vi "Dresden R2R Sputter 03.02.2018 IY24.vi"() -> ()   [LabVIEW 2009] (continued)
                                }
                                frame #1 {
                                }
                                }
                                }
                                frame #2 {
                                n31527 = local read "Semi"() -> (w36220:bool)
                                n31528 = case shown="False" w36220 {
                                frame #0 {
                                n31529 = local write "Dc_auto_set_zero"(TRUE ("Dc_auto_set")) -> ()
                                }
                                frame #1 {
                                }
                                }
                                }
                                frame #3 {
                                n31530 = local read "Semi"() -> (w36222:bool)
                                n31531 = case shown="False" w36222 {
                                frame #0 {
                                n31532 = Wait (ms)(milliseconds to wait=u32 1000) -> ()  [unwired: 1 out]
                                }
                                frame #1 {
                                }
                                }
                                }
                                frame #4 {
                                n31533 = local read "Semi"() -> (w36224:bool)
                                n31534 = case shown="False" w36224 {
                                frame #0 {
                                n31535 = while {
                                i -> [w36236]
                                stop <- w36225 stop-if-true
                                n31536 = Greater?(x=w36236, y=600) -> (0:w36235:bool)
                                n31537 = case shown="True" w36235 {
                                frame #0 {
                                }
                                frame #1 {
                                n31538 = local write "Semi"(TRUE ("Semi")) -> ()
                                n31539 = local write "Error Message"("Sputter Process cancelled.\nPlease Check DC connections." ("Error Message")) -> ()
                                }
                                }
                                n31540 = local read "Actual DC Power"() -> (w36230:dbl)
                                n31541 = local read "Actual DC Volt :"() -> (w36229:dbl)
                                n31542 = Less?(x=w36230, y=10.0) -> (x < y?=w36233:bool)
                                n31543 = Less?(x=w36229, y=20.0) -> (x < y?=w36234:bool)
                                n31544 = And(x=w36233, y=w36234) -> (x .and. y?=w36227:bool)
                                n31545 = local read "Semi"() -> (w36226:bool)
                                n31546 = Wait Until Next ms Multiple(millisecond multiple=u32 500) -> ()  [unwired: 1 out]
                                n31547 = Compound Arithmetic op=OR(w36227, w36226) -> (w36225:bool)
                                }
                                }
                                frame #1 {
                                }
                                }
                                }
                                frame #5 {
                                n31548 = local read "Semi"() -> (w36240:bool)
                                n31549 = case shown="False" w36240 {
                                frame #0 {
                                n31550 = while {
                                i -> [w36246]
                                stop <- w36241 stop-if-true
                                n31551 = Greater?(x=w36246, y=50) -> (0:w36245:bool)
                                n31552 = case shown="True" w36245 {
                                frame #0 {
                                }
                                frame #1 {
                                n31553 = local write "Semi"(TRUE ("Semi")) -> ()
                                n31554 = local write "Error Message"("Sputter Process cancelled.\nPlease Check DCPS-SW1." ("Error Message")) -> ()
                                }
                                }
                                n31555 = local read "Cnt_Dcps_sw1_di"() -> (w36244:bool)
                                n31556 = case shown="True" w36244 {
                                tunnel: [TRUE ("Cnt_Dcps_sw1_do") FALSE ("Cnt_Dcps_sw1_do")] -> w36243
                                frame #0 {
                                }
                                frame #1 {
                                n31557 = local write "Cnt_Dcps_sw1_do"(FALSE ("Cnt_Dcps_sw1_do")) -> ()
                                n31558 = Wait Until Next ms Multiple(millisecond multiple=u32 500) -> ()  [unwired: 1 out]
                                }
                                }
                                n31559 = local read "Semi"() -> (w36242:bool)
                                n31560 = Or(x=w36243, y=w36242) -> (x .or. y?=w36241:bool)
                                }
                                }
                                frame #1 {
                                }
                                }
                                }
                                frame #6 {
                                n31561 = local read "Semi"() -> (w36254:bool)
                                n31562 = case shown="False" w36254 {
                                frame #0 {
                                n31563 = Wait (ms)(milliseconds to wait=u32 1000) -> ()  [unwired: 1 out]
                                n31564 = local write "SDC1 25"(TRUE ("SDC1 25")) -> ()
                                }
                                frame #1 {
                                }
                                }
                                }
                                }
                                }
                                frame #1 {
                                }
                                }
                                }
                                frame #14 {
                                # "PC-BV OPEN"
                                n31565 = stacked-sequence {
                                frame #0 {
                                n31566 = local read "Semi"() -> (w36257:bool)
                                n31567 = case shown="False" w36257 {
                                frame #0 {
                                n31568 = stacked-sequence {
                                frame #0 {
                                n31569 = local read "Semi"() -> (w36258:bool)
                                n31570 = case shown="False" w36258 {
                                frame #0 {
                                n31571 = local write "Pc_bv2_auto_open"(TRUE ("Tp1_auto_start")) -> ()
                                }
                                frame #1 {
                                }
                                }
                                }
                                frame #1 {
                                n31572 = local read "Semi"() -> (w36260:bool)
                                n31573 = case shown="False" w36260 {
                                frame #0 {
                                n31574 = Wait (ms)(milliseconds to wait=u32 1000) -> ()  [unwired: 1 out]
                                }
                                frame #1 {
                                }
                                }
                                }
                                frame #2 {
                                n31575 = local read "Semi"() -> (w36262:bool)
                                n31576 = case shown="False" w36262 {
                                frame #0 {
                                n31577 = while {
                                i -> [w36268]
                                stop <- w36264 stop-if-true
                                n31578 = local read "Pc_bv_opened_ch2"() -> (w36266:bool)
                                n31579 = Greater?(x=w36268, y=120) -> (0:w36267:bool)
                                n31580 = local read "Semi"() -> (w36265:bool)
                                n31581 = Compound Arithmetic op=OR(w36265, w36266, w36267) -> (w36264:bool)
                                n31582 = Wait (ms)(milliseconds to wait=u32 500) -> ()  [unwired: 1 out]
                                }
                                }
                                frame #1 {
                                }
                                }
                                }
                                frame #3 {
                                n31583 = local read "Semi"() -> (w36270:bool)
                                n31584 = case shown="False" w36270 {
                                frame #0 {
                                n31585 = local read "Pc_bv_opened_ch2"() -> (w36271:bool)
                                n31586 = case shown="False" w36271 {
                                frame #0 {
                                n31587 = local write "Pc_bv2_auto_open"(TRUE ("Pc_bv1_auto_open")) -> ()
                                }
                                frame #1 {
                                }
                                }
                                }
                                frame #1 {
                                }
                                }
                                }
                                frame #4 {
                                n31588 = local read "Semi"() -> (w36273:bool)
                                n31589 = case shown="False" w36273 {
                                frame #0 {
                                n31590 = local read "Pc_bv_opened_ch2"() -> (w36274:bool)
                                n31591 = case shown="False" w36274 {
                                frame #0 {
                                n31592 = Wait (ms)(milliseconds to wait=u32 1000) -> ()  [unwired: 1 out]
                                }
                                frame #1 {
                                }
                                }
                                }
                                frame #1 {
                                }
                                }
                                }
                                frame #5 {
                                n31593 = local read "Semi"() -> (w36276:bool)
                                n31594 = case shown="False" w36276 {
                                frame #0 {
                                n31595 = while {
                                i -> [w36282]
                                stop <- w36278 stop-if-true
                                n31596 = local read "Pc_bv_opened_ch2"() -> (w36280:bool)
                                n31597 = Greater?(x=w36282, y=120) -> (0:w36281:bool)
                                n31598 = local read "Semi"() -> (w36279:bool)
                                n31599 = Compound Arithmetic op=OR(w36279, w36280, w36281) -> (w36278:bool)
                                n31600 = Wait (ms)(milliseconds to wait=u32 500) -> ()  [unwired: 1 out]
                                }
                                }
                                frame #1 {
                                }
                                }
                                }
                                frame #6 {
                                n31601 = local read "Semi"() -> (w36284:bool)
                                n31602 = case shown="False" w36284 {
                                frame #0 {
                                n31603 = local read "Pc_bv_opened_ch2"() -> (w36285:bool)
                                n31604 = case shown="False" w36285 {
                                frame #0 {
                                n31605 = local write "Error Message"("Start up process  cancelled\nbecause  PC-BV not opened.\nPlease check PC-BV1 connections." ("Error Message")) -> ()
                                n31606 = Wait (ms)(milliseconds to wait=u32 1000) -> ()  [unwired: 1 out]
                                }
                                frame #1 {
                                }
                                }
                                }
                                frame #1 {
                                }
                                }
                                }
                                }
                                }
                                frame #1 {
                                }
                                }
                                }
                                frame #1 {
                                n31607 = local read "Semi"() -> (w36288:bool)
                                n31608 = case shown="False" w36288 {
                                frame #0 {
                                n31609 = Wait (ms)(milliseconds to wait=u32 1000) -> ()  [unwired: 1 out]
                                n31610 = local write "SDC1 28"(TRUE ("SDC1 28")) -> ()
                                }
                                frame #1 {
                                }
                                }
                                }
                                }
                                }
                                frame #15 {
                                # "set ar zero"
                                n31611 = stacked-sequence {
                                frame #0 {
                                n31612 = local read "Semi"() -> (w36291:bool)
                                n31613 = case shown="False" w36291 {
                                frame #0 {
                                n31614 = stacked-sequence {
                                frame #0 {
                                n31615 = local read "Semi"() -> (w36292:bool)
                                n31616 = case shown="False" w36292 {
                                frame #0 {
                                n31617 = local write "Ar_auto_set_zero_ch2"(TRUE ("Ar_auto_set_zero_ch1")) -> ()
                                }
                                frame #1 {
                                }
                                }
                                }
                                frame #1 {
                                n31618 = local read "Semi"() -> (w36294:bool)
                                n31619 = case shown="False" w36294 {
                                frame #0 {
                                n31620 = while {
                                i -> [w36297]
                                stop <- w36296 stop-if-true
                                n31621 = Greater?(x=w36297, y=150) -> (0:w36296:bool)
                                n31622 = local read "Semi"() -> (w36295:bool)
                                n31623 = case shown="False" w36295 {
                                tunnel: [FALSE TRUE] -> _
                                frame #0 {
                                n31624 = Wait Until Next ms Multiple(millisecond multiple=u32 200) -> ()  [unwired: 1 out]
                                }
                                frame #1 {
                                }
                                }
                                }
                                }
                                frame #1 {
                                }
                                }
                                }
                                frame #2 {
                                n31625 = local read "Semi"() -> (w36302:bool)
                                n31626 = case shown="False" w36302 {
                                frame #0 {
                                n31627 = local read "Ar_sccm_act 6"() -> (w36304:dbl)
                                n31628 = Less?(x=w36304, y=1) -> (x < y?=w36303:bool)
                                n31629 = case shown="False" w36303 {
                                frame #0 {
                                n31630 = local write "Ar_auto_set_zero_ch2"(TRUE ("Ar_auto_set_zero_ch1")) -> ()
                                }
                                frame #1 {
                                }
                                }
                                }
                                frame #1 {
                                }
                                }
                                }
                                frame #3 {
                                n31631 = local read "Semi"() -> (w36307:bool)
                                n31632 = case shown="False" w36307 {
                                frame #0 {
                                n31633 = local read "Ar_sccm_act 6"() -> (w36309:dbl)
                                n31634 = Less?(x=w36309, y=1) -> (x < y?=w36308:bool)
                                n31635 = case shown="False" w36308 {
                                frame #0 {
                                n31636 = while {
                                i -> [w36315]
                                stop <- w36312 stop-if-true
                                n31637 = Greater?(x=w36315, y=150) -> (0:w36313:bool)
                                n31638 = local read "Semi"() -> (w36311:bool)
                                n31639 = case shown="True" w36311 {
                                tunnel: [FALSE FALSE] -> w36314
                                frame #0 {
                                }
                                frame #1 {
                                n31640 = Wait Until Next ms Multiple(millisecond multiple=u32 200) -> ()  [unwired: 1 out]
                                }
                                }
                                n31641 = Or(x=w36314, y=w36313) -> (x .or. y?=w36312:bool)
                                }
                                }
                                frame #1 {
                                }
                                }
                                }
                                frame #1 {
                                }
                                }
                                }
                                frame #4 {
                                n31642 = local read "Semi"() -> (w36320:bool)
                                n31643 = case shown="False" w36320 {
                                frame #0 {
                                n31644 = Wait (ms)(milliseconds to wait=u32 1000) -> ()  [unwired: 1 out]
                                }
                                frame #1 {
                                }
                                }
                                }
                                }
                                }
                                frame #1 {
                                }
                                }
                                }
                                frame #1 {
                                n31645 = local read "Semi"() -> (w36322:bool)
                                n31646 = case shown="False" w36322 {
                                frame #0 {
                                n31647 = local write "SDC1 26"(TRUE ("SDC1 26")) -> ()
                                n31648 = Wait (ms)(milliseconds to wait=u32 1000) -> ()  [unwired: 1 out]
                                }
                                frame #1 {
                                }
                                }
                                }
                                }
                                }
                                frame #16 {
                                # "sov-ar close"
                                n31649 = stacked-sequence {
                                frame #0 {
                                n31650 = local read "Semi"() -> (w36325:bool)
                                n31651 = case shown="False" w36325 {
                                frame #0 {
                                n31652 = while {
                                i -> [w36331]
                                stop <- w36326 stop-if-true
                                n31653 = Greater?(x=w36331, y=50) -> (0:w36330:bool)
                                n31654 = case shown="True" w36330 {
                                frame #0 {
                                }
                                frame #1 {
                                n31655 = local write "Semi"(TRUE ("Semi")) -> ()
                                n31656 = local write "Error Message"("Coating Process  \nwas cancelled.\nPlease check \nSOV-Ar connection." ("Error Message")) -> ()
                                }
                                }
                                n31657 = local read "Ch2_Sov_Ar_di"() -> (w36329:bool)
                                n31658 = case shown="True" w36329 {
                                tunnel: [TRUE FALSE] -> w36328
                                frame #0 {
                                }
                                frame #1 {
                                n31659 = local write "Ch2_Sov_Ar_do"(FALSE ("Ch1_WFC_do")) -> ()
                                n31660 = Wait Until Next ms Multiple(millisecond multiple=u32 200) -> ()  [unwired: 1 out]
                                }
                                }
                                n31661 = local read "Semi"() -> (w36327:bool)
                                n31662 = Or(x=w36328, y=w36327) -> (x .or. y?=w36326:bool)
                                }
                                }
                                frame #1 {
                                }
                                }
                                }
                                frame #1 {
                                n31663 = local read "Semi"() -> (w36339:bool)
                                n31664 = case shown="False" w36339 {
                                frame #0 {
                                n31665 = local write "SDC1 27"(TRUE ("SDC1 27")) -> ()
                                n31666 = Wait (ms)(milliseconds to wait=u32 1000) -> ()  [unwired: 1 out]
                                }
                                frame #1 {
                                }
                                }
                                }
                                }
                                }
                                frame #17 {
                                # "CC OPEN"
                                n31667 = stacked-sequence {
                                frame #0 {
                                n31668 = local read "Semi"() -> (w36342:bool)
                                n31669 = case shown="False" w36342 {
                                frame #0 {
                                n31670 = while {
                                i -> [w36348]
                                stop <- w36343 stop-if-true
                                n31671 = Greater?(x=w36348, y=50) -> (0:w36347:bool)
                                n31672 = case shown="True" w36347 {
                                frame #0 {
                                }
                                frame #1 {
                                n31673 = local write "Semi"(TRUE ("Semi")) -> ()
                                n31674 = local write "Error Message"("Coating Process  \nwas cancelled.\nPlease check \nBG-BV connection." ("Error Message")) -> ()
                                }
                                }
                                n31675 = local read "Ch2_Cc_on_off_di"() -> (w36346:bool)
                                n31676 = case shown="False" w36346 {
                                tunnel: [FALSE TRUE] -> w36345
                                frame #0 {
                                n31677 = local write "Ch2_Cc_on_off_do"(TRUE ("Ch1_WFC_do")) -> ()
                                n31678 = Wait Until Next ms Multiple(millisecond multiple=u32 200) -> ()  [unwired: 1 out]
                                }
                                frame #1 {
                                }
                                }
                                n31679 = local read "Semi"() -> (w36344:bool)
                                n31680 = Or(x=w36345, y=w36344) -> (x .or. y?=w36343:bool)
                                }
                                }
                                frame #1 {
                                }
                                }
                                }
                                frame #1 {
                                n31681 = local read "Semi"() -> (w36356:bool)
                                n31682 = case shown="False" w36356 {
                                frame #0 {
                                n31683 = while {
                                i -> [w36361]
                                stop <- w36359 stop-if-true
                                n31684 = Greater?(x=w36361, y=30) -> (0:w36357:bool)
                                n31685 = Wait Until Next ms Multiple(millisecond multiple=u32 1000) -> ()  [unwired: 1 out]
                                n31686 = local read "Semi"() -> (w36360:bool)
                                n31687 = Or(x=w36357, y=w36360) -> (x .or. y?=w36359:bool)
                                }
                                }
                                frame #1 {
                                }
                                }
                                }
                                frame #2 {
                                n31688 = local read "Semi"() -> (w36363:bool)
                                n31689 = case shown="False" w36363 {
                                frame #0 {
                                n31690 = local write "SDC1 27b"(TRUE ("SDC1 3")) -> ()
                                n31691 = Wait (ms)(milliseconds to wait=u32 1000) -> ()  [unwired: 1 out]
                                }
                                frame #1 {
                                }
                                }
                                }
                                }
                                }
                                frame #18 {
                                # "CHECK CHAMBER PRESSURE"
                                n31692 = stacked-sequence {
                                frame #0 {
                                n31693 = local read "Semi"() -> (w36366:bool)
                                n31694 = case shown="False" w36366 {
                                frame #0 {
                                n31695 = while {
                                i -> [w36374]
                                stop <- w36368 stop-if-true
                                n31696 = Greater?(x=w36374, y=300) -> (0:w36373:bool)
                                n31697 = case shown="True" w36373 {
                                frame #0 {
                                }
                                frame #1 {
                                n31698 = local write "Semi"(TRUE ("Semi")) -> ()
                                n31699 = local write "Error Message"("Coating Process cancelled.\nPlease check chamber \nconnections." ("Error Message")) -> ()
                                }
                                }
                                n31700 = local read "Ch_CC_press_ch2 2"() -> (w36367:dbl)
                                n31701 = Greater Or Equal?(x=w36367, y=5e-05 ("CHAMBER PRESSURE 6")) -> (x >= y?=w36371:bool)
                                n31702 = case shown="True" w36371 {
                                tunnel: [TRUE FALSE] -> w36370
                                frame #0 {
                                }
                                frame #1 {
                                n31703 = Wait Until Next ms Multiple(millisecond multiple=u32 200) -> ()  [unwired: 1 out]
                                }
                                }
                                n31704 = local read "Semi"() -> (w36369:bool)
                                n31705 = Or(x=w36370, y=w36369) -> (x .or. y?=w36368:bool)
                                }
                                }
                                frame #1 {
                                }
                                }
                                }
                                frame #1 {
                                n31706 = local read "Semi"() -> (w36381:bool)
                                n31707 = case shown="False" w36381 {
                                frame #0 {
                                n31708 = Wait (ms)(milliseconds to wait=u32 1000) -> ()  [unwired: 1 out]
                                n31709 = local write "SDC1 27c"(TRUE ("SDC1 10")) -> ()
                                }
                                frame #1 {
                                }
                                }
                                }
                                }
                                }
                                frame #19 {
                                n31710 = local read "Semi"() -> (w36384:bool)
                                n31711 = case shown="False" w36384 {
                                frame #0 {
                                n31712 = Wait (ms)(milliseconds to wait=u32 2500) -> ()  [unwired: 1 out]
                                n31713 = local write "Cnt_Do_Buzzer"(TRUE ("SDC1 30")) -> ()
                                n31714 = local write "SDC1 30"(TRUE ("SDC1 30")) -> ()
                                }
                                frame #1 {
                                }
                                }
                                }
                                frame #20 {
                                n31715 = local read "Semi"() -> (w36388:bool)
                                n31716 = case shown="False" w36388 {
                                frame #0 {
                                n31717 = Wait (ms)(milliseconds to wait=u32 1000) -> ()  [unwired: 1 out]
                                n31718 = local write "Cnt_Do_Buzzer"(FALSE ("SDC1 30")) -> ()
                                }
                                frame #1 {
                                }
                                }
                                }
                                }
                                }
                                frame #1 {
                                }
                                }
                                }
                                }
                                }
                                frame #3 {
                                n31719 = stacked-sequence {
                                frame #0 {
                                n31720 = local write "Transfer_ch2_3"(TRUE ("Transfer_ch3_2")) -> ()
                                n31721 = Wait (ms)(milliseconds to wait=u32 100) -> ()  [unwired: 1 out]
                                }
                                frame #1 {
                                n31722 = while {
                                stop <- w36394 stop-if-true
                                n31723 = Wait Until Next ms Multiple(millisecond multiple=u32 300) -> ()  [unwired: 1 out]
                                n31724 = local read "Transfer_ch2_3"() -> (w36395:bool)
                                n31725 = local read "Semi"() -> (w36397:bool)
                                n31726 = Not(x=w36395) -> (.not. x?=w36396:bool)
                                n31727 = Or(x=w36396, y=w36397) -> (x .or. y?=w36394:bool)
                                }
                                }
                                }
                                }
                                }
                                }
                                frame #1 {
                                }
                                }
                                n31728 = local read "Semi"() -> (w34613:bool)
                                n31729 = Or(x=w34609, y=w34613) -> (x .or. y?=w34612:bool)
                              }
                            }
                            frame #1 {
                              n31730 = disable-structure shown="Disabled" {
                                frame #0 {
                                n31731 = local read "Single_ch3_Interlock"() -> (w36399:dbl)
                                n31732 = local read "Ch3_pressure"() -> (w36403:dbl)
                                n31733 = local read "started_up_ch3"() -> (w36401:bool)
                                n31734 = In Range and Coerce(upper limit=w36399, x=w36403, lower limit=1e-08) -> (In Range?=w36404:bool)  [unwired: 1 out]
                                n31735 = And(x=w36404, y=w36401) -> (x .and. y?=w36400:bool)
                                n31736 = case shown="True" w36400 {
                                frame #0 {
                                }
                                frame #1 {
                                n31737 = local read "Semi"() -> (w36405:bool)
                                n31738 = case shown="False" w36405 {
                                frame #0 {
                                n31739 = stacked-sequence {
                                frame #0 {
                                # "WATER FLOW CONTROL OPEN"
                                n31740 = stacked-sequence {
                                frame #0 {
                                n31741 = local read "Semi"() -> (w36406:bool)
                                n31742 = case shown="False" w36406 {
                                frame #0 {
                                n31743 = while {
                                i -> [w36412]
                                stop <- w36407 stop-if-true
                                n31744 = Greater?(x=w36412, y=100) -> (0:w36411:bool)
                                n31745 = case shown="True" w36411 {
                                frame #0 {
                                }
                                frame #1 {
                                n31746 = local write "Semi"(TRUE ("Semi")) -> ()
                                n31747 = local write "Error Message"("Coating Process  \nwas cancelled.\nPlease check water \nflow connection." ("Error Message")) -> ()
                                }
                                }
                                n31748 = local read "Ch4_WFS_di"() -> (w36410:bool)
                                n31749 = case shown="True" w36410 {
                                tunnel: [TRUE FALSE] -> w36409
                                frame #0 {
                                }
                                frame #1 {
                                n31750 = local write "Ch4_WFC_do"(FALSE ("Ch1_WFC_do")) -> ()
                                n31751 = Wait Until Next ms Multiple(millisecond multiple=u32 200) -> ()  [unwired: 1 out]
                                }
                                }
                                n31752 = local read "Semi"() -> (w36408:bool)
                                n31753 = Or(x=w36409, y=w36408) -> (x .or. y?=w36407:bool)
                                }
                                }
                                frame #1 {
                                }
                                }
                                }
                                frame #1 {
                                n31754 = local read "Semi"() -> (w36420:bool)
                                n31755 = case shown="False" w36420 {
                                frame #0 {
                                n31756 = while {
                                i -> [w36426]
                                stop <- w36421 stop-if-true
                                n31757 = Greater?(x=w36426, y=100) -> (0:w36425:bool)
                                n31758 = case shown="True" w36425 {
                                frame #0 {
                                }
                                frame #1 {
                                n31759 = local write "Semi"(TRUE ("Semi")) -> ()
                                n31760 = local write "Error Message"("Coating Process  \nwas cancelled.\nPlease check water \nflow connection." ("Error Message")) -> ()
                                }
                                }
                                n31761 = local read "Ch1_WFS_di"() -> (w36424:bool)
                                n31762 = case shown="True" w36424 {
                                tunnel: [TRUE FALSE] -> w36423
                                frame #0 {
                                }
                                frame #1 {
                                n31763 = local write "Ch1_WFC_do"(FALSE ("Ch1_WFC_do")) -> ()
                                n31764 = Wait Until Next ms Multiple(millisecond multiple=u32 200) -> ()  [unwired: 1 out]
                                }
                                }
                                n31765 = local read "Semi"() -> (w36422:bool)
                                n31766 = Or(x=w36423, y=w36422) -> (x .or. y?=w36421:bool)
                                }
                                }
                                frame #1 {
                                }
                                }
                                }
                                frame #2 {
                                n31767 = local read "Semi"() -> (w36434:bool)
                                n31768 = case shown="False" w36434 {
                                frame #0 {
                                n31769 = while {
                                i -> [w36440]
                                stop <- w36435 stop-if-true
                                n31770 = Greater?(x=w36440, y=100) -> (0:w36439:bool)
                                n31771 = case shown="True" w36439 {
                                frame #0 {
                                }
                                frame #1 {
                                n31772 = local write "Semi"(TRUE ("Semi")) -> ()
                                n31773 = local write "Error Message"("Coating Process  \nwas cancelled.\nPlease check water \nflow connection." ("Error Message")) -> ()
                                }
                                }
                                n31774 = local read "Ch2_WFS_di"() -> (w36438:bool)
                                n31775 = case shown="True" w36438 {
                                tunnel: [TRUE FALSE] -> w36437
                                frame #0 {
                                }
                                frame #1 {
                                n31776 = local write "Ch2_WFC_do"(FALSE ("Ch1_WFC_do")) -> ()
                                n31777 = Wait Until Next ms Multiple(millisecond multiple=u32 200) -> ()  [unwired: 1 out]
                                }
                                }
                                n31778 = local read "Semi"() -> (w36436:bool)
                                n31779 = Or(x=w36437, y=w36436) -> (x .or. y?=w36435:bool)
                                }
                                }
                                frame #1 {
                                }
                                }
                                }
                                frame #3 {
                                n31780 = local read "Semi"() -> (w36448:bool)
                                n31781 = case shown="False" w36448 {
                                frame #0 {
                                n31782 = while {
                                i -> [w36454]
                                stop <- w36449 stop-if-true
                                n31783 = Greater?(x=w36454, y=100) -> (0:w36453:bool)
                                n31784 = case shown="True" w36453 {
                                frame #0 {
                                }
                                frame #1 {
                                n31785 = local write "Semi"(TRUE ("Semi")) -> ()
                                n31786 = local write "Error Message"("Coating Process  \nwas cancelled.\nPlease check water \nflow connection." ("Error Message")) -> ()
                                }
                                }
                                n31787 = local read "Ch3_WFS_di"() -> (w36452:bool)
                                n31788 = case shown="False" w36452 {
                                tunnel: [FALSE TRUE] -> w36451
                                frame #0 {
                                n31789 = local write "Ch3_WFC_do"(TRUE ("Ch1_WFC_do")) -> ()
                                n31790 = Wait Until Next ms Multiple(millisecond multiple=u32 200) -> ()  [unwired: 1 out]
                                }
                                frame #1 {
                                }
                                }
                                n31791 = local read "Semi"() -> (w36450:bool)
                                n31792 = Or(x=w36451, y=w36450) -> (x .or. y?=w36449:bool)
                                }
                                }
                                frame #1 {
                                }
                                }
                                }
                                frame #4 {
                                n31793 = local read "Semi"() -> (w36462:bool)
                                n31794 = case shown="False" w36462 {
                                frame #0 {
                                n31795 = local write "SDC1 2"(TRUE ("SDC1 2")) -> ()
                                n31796 = Wait (ms)(milliseconds to wait=u32 1000) -> ()  [unwired: 1 out]
                                }
                                frame #1 {
                                }
                                }
                                }
                                }
                                }
                                frame #1 {
                                # "BG-BV open"
                                n31797 = stacked-sequence {
                                frame #0 {
                                n31798 = local read "Semi"() -> (w36465:bool)
                                n31799 = case shown="False" w36465 {
                                frame #0 {
                                n31800 = while {
                                i -> [w36471]
                                stop <- w36466 stop-if-true
                                n31801 = Greater?(x=w36471, y=50) -> (0:w36470:bool)
                                n31802 = case shown="True" w36470 {
                                frame #0 {
                                }
                                frame #1 {
                                n31803 = local write "Semi"(TRUE ("Semi")) -> ()
                                n31804 = local write "Error Message"("Coating Process  \nwas cancelled.\nPlease check \nBG-BV connection." ("Error Message")) -> ()
                                }
                                }
                                n31805 = local read "Ch3_Bg_bv_di"() -> (w36469:bool)
                                n31806 = case shown="False" w36469 {
                                tunnel: [FALSE TRUE] -> w36468
                                frame #0 {
                                n31807 = local write "Ch3_Bg_bv_do"(TRUE ("Ch1_WFC_do")) -> ()
                                n31808 = Wait Until Next ms Multiple(millisecond multiple=u32 200) -> ()  [unwired: 1 out]
                                }
                                frame #1 {
                                }
                                }
                                n31809 = local read "Semi"() -> (w36467:bool)
                                n31810 = Or(x=w36468, y=w36467) -> (x .or. y?=w36466:bool)
                                }
                                }
                                frame #1 {
                                }
                                }
                                }
                                frame #1 {
                                n31811 = local read "Semi"() -> (w36479:bool)
                                n31812 = case shown="False" w36479 {
                                frame #0 {
                                n31813 = Wait (ms)(milliseconds to wait=u32 1000) -> ()  [unwired: 1 out]
                                n31814 = local write "SDC1 4"(TRUE ("SDC1 4")) -> ()
                                }
                                frame #1 {
                                }
                                }
                                }
                                }
                                }
                                frame #2 {
                                # "Baratron set zero"
                                n31815 = stacked-sequence {
                                frame #0 {
                                n31816 = local write "Pc_bv3_auto_baratron_set_zero"(TRUE ("Pc_bv2_auto_baratron_set_zero")) -> ()